vi "UHR-Fleezers Control (host) - 12.3.1.vi"() -> ()   [LabVIEW 2012] (continued)
        n2497 = Add(x=w3700, y=w3699) -> (x+y=w3686:dbl[][])
        n2498 = Add(x=w3674, y=w3673) -> (x+y=w3660:dbl[][])
        n2499 = Add(x=w3768, y=w3767) -> (x+y=w3766:dbl[][])
        n2500 = Add(x=w3772, y=w3771) -> (x+y=w3746:dbl[][])
        n2501 = Add(x=w3754, y=w3753) -> (x+y=w3752:dbl[][])
        n2502 = Add(x=w3761, y=w3760) -> (x+y=w3759:dbl[][])
        n2503 = Divide(x=w3752, y=2) -> (x/y=w3750:dbl[][])
        n2504 = Divide(x=w3766, y=2) -> (x/y=w3711:dbl[][])
        n2505 = To Single Precision Float(number=w3746) -> (single precision float=w3745:sgl[][])
        n2506 = To Single Precision Float(number=w3686) -> (single precision float=w3690:sgl[][])
        n2507 = To Single Precision Float(number=w3660) -> (single precision float=w3664:sgl[][])
        n2508 = Divide(x=w3759, y=2) -> (x/y=w3713:dbl[][])
        n2509 = Transpose 2D Array(2D array=w3750) -> (transposed array=→"Data map":dbl[][])
        n2510 = To Single Precision Float(number=w3711) -> (single precision float=w3717:sgl[][])
        n2511 = To Single Precision Float(number=w3713) -> (single precision float=w3714:sgl[][])
        n2512 = call "IMAQ ArrayToImage"("Image Pixels (Float)"=w3745, "Image"=w3683) -> ("Image Out"=w3748:T2)  [unwired: 8 in, 1 out]
        n2513 = call "IMAQ ArrayToImage"("Image Pixels (Float)"=w3690, "Image"=w3682) -> ("Image Out"=w3692:T2)  [unwired: 8 in, 1 out]
        n2514 = call "IMAQ ArrayToImage"("Image Pixels (Float)"=w3664, "Image"=w3656) -> ("Image Out"=w3666:T2)  [unwired: 8 in, 1 out]
        n2515 = call "IMAQ ArrayToImage"("Image Pixels (Float)"=w3717, "Image"=w3657) -> ("Image Out"=w3719:T2)  [unwired: 8 in, 1 out]
        n2516 = call "IMAQ Symmetry"("Type of Symmetry"=w3747, "Image Src"=w3748) -> ("Image Dst Out"=w3743:T2)  [unwired: 3 in, 1 out]
        n2517 = call "IMAQ ArrayToImage"("Image Pixels (Float)"=w3714, "Image"=w3658) -> ("Image Out"=w3716:T2)  [unwired: 8 in, 1 out]
        n2518 = call "IMAQ Symmetry"("Type of Symmetry"=w3691, "Image Src"=w3692) -> ("Image Dst Out"=w3688:T2)  [unwired: 3 in, 1 out]
        n2519 = call "IMAQ Symmetry"("Type of Symmetry"=w3665, "Image Src"=w3666) -> ("Image Dst Out"=w3662:T2)  [unwired: 3 in, 1 out]
        n2520 = call "IMAQ Symmetry"("Type of Symmetry"=w3718, "Image Src"=w3719) -> ("Image Dst Out"=→"Detection Laser X":T2)  [unwired: 3 in, 1 out]
        n2521 = call "IMAQ Symmetry"("Type of Symmetry"=w3715, "Image Src"=w3716) -> ("Image Dst Out"=→"Detection Laser Y":T2)  [unwired: 3 in, 1 out]
        n2522 = call "IMAQ Set Simple Calibration"("Calibration Axis Info"=T33 {"Origin Pixel"={"X"=0.0, "Y"=0.0}, "Angle Relative to Horizontal (deg)"=0.0, "Axis Reference"=0}, "Grid Descriptor"=T34 {"X Step"=0.3, "Y Step"=0.3, "Unit"=enum."Undefined"}, "Image"=w3743) -> ("Calibrated Image"=→"APD 1":T2)  [unwired: 7 in, 1 out]
        n2523 = call "IMAQ Set Simple Calibration"("Calibration Axis Info"=T33 {"Origin Pixel"={"X"=0.0, "Y"=0.0}, "Angle Relative to Horizontal (deg)"=0.0, "Axis Reference"=0}, "Grid Descriptor"=T34 {"X Step"=0.3, "Y Step"=0.3, "Unit"=enum."Undefined"}, "Image"=w3688) -> ("Calibrated Image"=→"APD 2":T2)  [unwired: 7 in, 1 out]
        n2524 = call "IMAQ Set Simple Calibration"("Calibration Axis Info"=T33 {"Origin Pixel"={"X"=0.0, "Y"=0.0}, "Angle Relative to Horizontal (deg)"=0.0, "Axis Reference"=0}, "Grid Descriptor"=T34 {"X Step"=0.3, "Y Step"=0.3, "Unit"=enum."Undefined"}, "Image"=w3662) -> ("Calibrated Image"=→"APD 3":T2)  [unwired: 7 in, 1 out]
      }
    }
    n2525 = case "For computing FFTs for display" shown="True" "Compute FFT" {
      tunnel: w3158 -> [_ w4286]
      frame False {
      }
      frame True {
        n2526 = Build Array("FFT 1 Choice 1", "FFT 1 Choice 2", "FFT 2 Choice 1", "FFT 2 Choice 2") -> (w4279:u16[])
        n2527 = Array Size(array=w4286) -> (size(s)=w4285:i32)
        n2528 = feedback-in #17(w4279) -> ()
        n2529 = feedback #17(u16[] [100, 100, 100, 100]) -> (w4280:u16[])
        n2530 = feedback-in #18("# Spectra to Ave.") -> ()
        n2531 = feedback #18("# Spectra to Ave.") -> (w4277:dbl)
        n2532 = Not Equal?(x="# Spectra to Ave.", y=w4277) -> (x != y?=w4276:bool)
        n2533 = Not Equal?(x=w4279, y=w4280) -> (x != y?=w4278:bool)
        n2534 = feedback #19(1.0) -> (w4263:dbl)
        n2535 = Compound Arithmetic op=OR("Reset FFT", w4278, w4276) -> (w4261:bool)
        n2536 = Select(t=1.0, s=w4261, f=w4263) -> (s? t:f=w4265:dbl)
        n2537 = Greater?(x=w4265, y="# Spectra to Ave.") -> (0:w4284:bool)
        n2538 = Increment(x=w4265) -> (x+1=w4264:dbl)
        n2539 = feedback-in #19(w4264) -> ()
        n2540 = local read "DMA Update Period (s)"() -> (w4259:dbl)
        n2541 = Multiply(x="# Spectra to Ave.", y=w4259) -> (x*y=→"Ave. Time (s)":dbl)
        n2542 = Build Array(cluster{"f0":dbl, "df":dbl, "magnitude":dbl[]} {"f0"=0.0, "df"=0.0, "magnitude"=[]} ("PSD")) -> (w4268:cluster{"f0":dbl, "df":dbl, "magnitude":dbl[]}[])
        n2543 = Build Array(w4268, w4268, w4268, w4268) -> (w4270:T43)
        n2544 = feedback #20(w4270) -> (w4275:T43)
        n2545 = for {
          N: 4 -> [_]
          tunnel: w4279 -> [w4308] mode=indexing
          tunnel: w4286 -> [w4309]
          tunnel: w4285 -> [w4311]
          tunnel: w4261 -> [w4304]
          tunnel: w4284 -> [w4303]
          tunnel: "# Spectra to Ave." -> [w4302]
          tunnel: [w4301] -> w4274 mode=indexing
          tunnel: w4275 -> [w4306] mode=indexing
          tunnel: [w4305] -> w4262 mode=indexing
          tunnel: w4265 -> [w4300]
          n2546 = Less?(x=w4308, y=w4311) -> (x < y?=w4310:bool)
          n2547 = Index Array(array=w4309, index=w4308) -> (element=w4307:waveform(dbl))
          n2548 = case shown="True" w4310 {
            tunnel: w4307 -> [_ w4328]
            tunnel: w4306 -> [w4313 w4326]
            tunnel: [w4313 w4314] -> w4305
            tunnel: w4304 -> [_ w4325]
            tunnel: w4303 -> [_ w4318]
            tunnel: w4302 -> [_ w4317]
            tunnel: [cluster{"f0":dbl, "df":dbl, "magnitude":dbl[]} {"f0"=0.0, "df"=0.0, "magnitude"=[]} ("PSD") w4319] -> w4301
            tunnel: w4300 -> [_ w4316]
            frame False {
            }
            frame True {
              n2549 = call <vilib>:"Std Deviation and Variance.vi"("X"=w4328) -> ("mean"=w4329:dbl)  [unwired: 1 in, 2 out]
              n2550 = Subtract(x=w4328, y=w4329) -> (x-y=w4327:waveform(dbl))
              n2551 = xnode "Spectral Measurements"("Signals"=w4327) -> ("PSD"=w4321:cluster{"f0":dbl, "df":dbl, "magnitude":dbl[]})  [unwired: 1 in, 1 out]
              n2552 = case shown="False" w4325 {
                tunnel: w4326 -> [w4338 _]
                tunnel: [w4334 w4343] -> w4314
                tunnel: w4321 -> [w4337 w4344]
                tunnel: w4318 -> [w4336 _]
                frame False {
                  n2553 = Build Array (concatenate)(w4338, w4337) -> (w4335:cluster{"f0":dbl, "df":dbl, "magnitude":dbl[]}[])
                  n2554 = case shown="True" w4336 {
                    tunnel: w4335 -> [w4339 w4342]
                    tunnel: [w4339 w4340] -> w4334
                    frame False {
                    }
                    frame True {
                      n2555 = Delete From Array(array=w4342, index=0) -> (array with subset deleted=w4340:cluster{"f0":dbl, "df":dbl, "magnitude":dbl[]}[])  [unwired: 1 in, 1 out]
                    }
                  }
                }
                frame True {
                  n2556 = Build Array(w4344) -> (w4343:cluster{"f0":dbl, "df":dbl, "magnitude":dbl[]}[])
                }
              }
              n2557 = for {
                tunnel: w4314 -> [w4333] mode=indexing
                tunnel: [w4332] -> w4324 mode=indexing
                workers-P: _ -> [_]
                n2558 = Unbundle By Name(w4333) -> ("magnitude"=w4332:dbl[])
              }
              n2559 = Transpose 2D Array(2D array=w4324) -> (transposed array=w4323:dbl[][])
              n2560 = for {
                tunnel: w4323 -> [w4331] mode=indexing
                tunnel: [w4330] -> w4322 mode=indexing
                workers-P: _ -> [_]
                n2561 = Add Array Elements(numeric array=w4331) -> (sum=w4330:dbl)
              }
              n2562 = Select(t=w4317, s=w4318, f=w4316) -> (s? t:f=w4315:dbl)
              n2563 = Divide(x=w4322, y=w4315) -> (x/y=w4320:dbl[])
              n2564 = Bundle By Name(cluster=w4321, "magnitude"=w4320) -> (w4319:cluster{"f0":dbl, "df":dbl, "magnitude":dbl[]})
            }
          }
        }
        n2565 = case shown="True" w4261 {
          tunnel: w4262 -> [w4293 w4299]
          tunnel: [w4293 w4294] -> w4260
          frame False {
          }
          frame True {
            n2566 = Array Subset(array=w4299, index (row)=0 ("index"), length (row)=4 ("length"), index (col)=0 ("index"), length (col)=1 ("length")) -> (w4294:T43)
          }
        }
        n2567 = feedback-in #20(w4260) -> ()
        n2568 = Split 1D Array(array=w4274, index=2) -> (first subarray=→"FFT 1":cluster{"f0":dbl, "df":dbl, "magnitude":dbl[]}[], second subarray=→"FFT 2":cluster{"f0":dbl, "df":dbl, "magnitude":dbl[]}[])
      }
    }
    n2569 = Index Array(array=w3156, index=4) -> (element=w3212:waveform(dbl))
    n2570 = Index Array(array=w3156, index=7) -> (element=w3209:waveform(dbl))
    n2571 = Divide(x="T1 offset_x (mV)", y=1000.0) -> (x/y=w3213:dbl)
    n2572 = feedback-in #21("Calibration") -> ()
    n2573 = feedback #21(u16 1 ("Calibration")) -> (w3231:u16)
    n2574 = Divide(x="T2 offset_x (mV)", y=1000.0) -> (x/y=w3211:dbl)
    n2575 = case shown="2" "Calibration" {
      tunnel: "T1 alpha_x (nm/V)" -> [_ w3607 w3628]
      tunnel: "T1 kappa_x (pN/nm)" -> [_ _ w3618]
      tunnel: "T2 alpha_x (nm/V)" -> [_ w3606 w3626]
      tunnel: "T2 kappa_x (pN/nm)" -> [_ _ w3619]
      tunnel: w3212 -> [w3589 w3604 w3624]
      tunnel: w3209 -> [w3588 w3602 w3622]
      tunnel: [w3589 w3601 w3621] -> w3240
      tunnel: [w3588 w3600 w3620] -> w3239
      tunnel: ["T1 X (V)" ("Label.Text") "T1 X (nm)" ("Label.Text") "T1 X (pN)" ("Label.Text")] -> w3228
      tunnel: ["T2 X (V)" ("Label.Text") "T2 X (nm)" ("Label.Text") "T2 X (pN)" ("Label.Text")] -> w3227
      tunnel: ["Position (V)" ("Label.Text") "Position (nm)" ("Label.Text") "Force (pN)" ("Label.Text")] -> w3229
      tunnel: w3211 -> [_ w3592 w3611]
      tunnel: w3213 -> [_ w3595 w3613]
      tunnel: ["Mean (V)" ("Label.Text") "Mean (nm)" ("Label.Text") "Mean (pN)" ("Label.Text")] -> w3224
      tunnel: ["Difference (V)" ("Label.Text") "Difference (nm)" ("Label.Text") "Difference (pN)" ("Label.Text")] -> w3164
      frame 0, Default {
      }
      frame 1 {
        n2576 = Unbundle By Name(w3604) -> ("Y"=w3608:dbl[])
        n2577 = Unbundle By Name(w3602) -> ("Y"=w3593:dbl[])
        n2578 = Subtract(x=w3608, y=w3595) -> (x-y=w3596:dbl[])
        n2579 = Subtract(x=w3593, y=w3592) -> (x-y=w3594:dbl[])
        n2580 = Multiply(x=w3594, y=w3606) -> (x*y=w3603:dbl[])
        n2581 = Multiply(x=w3607, y=w3596) -> (x*y=w3605:dbl[])
        n2582 = Bundle By Name(cluster=w3602, "Y"=w3603) -> (w3600:waveform(dbl))
        n2583 = Bundle By Name(cluster=w3604, "Y"=w3605) -> (w3601:waveform(dbl))
      }
      frame 2 {
        n2584 = Unbundle By Name(w3624) -> ("Y"=w3629:dbl[])
        n2585 = Unbundle By Name(w3622) -> ("Y"=w3627:dbl[])
        n2586 = Subtract(x=w3627, y=w3611) -> (x-y=w3612:dbl[])
        n2587 = Subtract(x=w3629, y=w3613) -> (x-y=w3614:dbl[])
        n2588 = Compound Arithmetic op=MULTIPLY(w3612, w3626, w3619) -> (w3623:dbl[])
        n2589 = Compound Arithmetic op=MULTIPLY(w3618, w3628, w3614) -> (w3625:dbl[])
        n2590 = Bundle By Name(cluster=w3622, "Y"=w3623) -> (w3620:waveform(dbl))
        n2591 = Bundle By Name(cluster=w3624, "Y"=w3625) -> (w3621:waveform(dbl))
      }
    }
    n2592 = case shown="True" "Read Lateness and Rel Phase" {
      tunnel: w3030 -> [w3538 w3577]
      tunnel: w3029 -> [w3539 w3576]
      tunnel: [w3538 w3543] -> w3206
      tunnel: [w3539 w3542] -> w3205
      frame False {
      }
      frame True {
        n2593 = xnode "Read/Write Control"("FPGA VI Reference In"=w3577, "error in"=w3576) -> ("FPGA VI Reference Out"=w3545:T19, "error out"=w3544:errorcluster, "GI Relative phase"=→"GI relative phase":i16, "Relative phase"=→"Relative phase (AI1)":i16, "AI Late Counter"=→"Late Counter (AI1)":u8, "GI Late Counter"=→"GI Late Counter":u8, "MCL Late Counter"=→"MCL Late Counter":u8, "MCL Relative Phase"=→"Relative Phase (MCL)":i16, "APD Acq Relative Phase"=→"APD Acq Relative Phase":i16, "APD 1 Gate Relative Phase"=→"APD 1 Gate Relative Phase":i16, "APD 2 Gate Relative Phase"=→"APD 2 Gate Relative Phase":i16, "APD Acq Late Counter"=→"APD Acq Late Counter":u8, "APD 1 Gate Late Counter"=→"APD 1 Gate Late Counter":u8, "APD 2 Gate Late Counter"=→"APD 2 Gate Late Counter":u8, "Green FB Relative Phase"=→"Relative phase (Green FB)":i16, "GI Relative phase 2"=→"GI relative phase 2":i16, "GI Late Counter 2"=→"GI Late Counter 2":u8, "Trap Pos FIFO Timeout"=→"Trap Pos FIFO Timeout":u16, "Trap AI FIFO Timeout"=→"Trap AI FIFO Timeout":u16, "RI Late Counter"=→"RI Late Counter":u8, "RI Late Counter 2"=→"RI Late Counter 2":u8, "RI Relative phase"=→"RI relative phase":i16, "RI Relative phase 2"=→"RI relative phase 2":i16, "Red FB Relative Phase"=→"Relative phase (RI FB)":i16, "Red Late Counter"=→"Red AI Late Counter":u8, "Green Late Counter"=→"Green AI Late Counter":u8, "BI Late Counter (AO)"=→"Late Counter (BI AO)":u8, "Blue Late Counter (D)"=→"Late Counter (BI DO)":u8, "Blue Int Late Counter"=→"Late Counter (BI AI)":u8, "Blue Int Relative Phase"=→"Relative phase (BI AI)":i16, "BI Relative phase (AO)"=→"Relative phase (BI AO)":i16, "BI Relative phase (D)"=→"Relative phase (BI DO)":i16)
        n2594 = xnode "Read/Write Control"("FPGA VI Reference In"=w3545, "error in"=w3544) -> ("FPGA VI Reference Out"=w3543:T19, "error out"=w3542:errorcluster, "APD 3 Gate Late Counter"=→"APD 3 Gate Late Counter":u8, "APD 3 Gate Relative Phase"=→"APD 3 Gate Relative Phase":i16)
      }
    }
    n2595 = Not Equal?(x=w3231, y="Calibration") -> (x != y?=w3190:bool)
    n2596 = case shown="True" w3190 {
      tunnel: w3229 -> [_ w3582]
      tunnel: w3228 -> [_ w3581]
      tunnel: w3227 -> [_ w3580]
      tunnel: w3224 -> [_ w3579]
      tunnel: w3164 -> [_ w3578]
      frame False {
      }
      frame True {
        n2597 = property on="Force" class="WFChart (strict)"("YScale.NameLbl.Text"=w3582) -> ()  [unwired: 2 in, 2 out]
        n2598 = property on="T2 X" class="DigNum (strict)"("Caption.Text"=w3580) -> ()  [unwired: 2 in, 2 out]
        n2599 = property on="T1 X" class="DigNum (strict)"("Caption.Text"=w3581) -> ()  [unwired: 2 in, 2 out]
        n2600 = property on="Mean" class="DigNum (strict)"("Caption.Text"=w3579) -> ()  [unwired: 2 in, 2 out]
        n2601 = property on="Difference" class="DigNum (strict)"("Caption.Text"=w3578) -> ()  [unwired: 2 in, 2 out]
      }
    }
    n2602 = Unbundle By Name(w3212) -> ("Y"=w3215:dbl[])
    n2603 = Unbundle By Name(w3209) -> ("Y"=w3218:dbl[])
    n2604 = Subtract(x=w3215, y=w3213) -> (x-y=w3216:dbl[])
    n2605 = Subtract(x=w3218, y=w3211) -> (x-y=w3217:dbl[])
    n2606 = Multiply(x=w3217, y="T2 alpha_x (nm/V)") -> (x*y=w3012:dbl[])
    n2607 = Multiply(x="T1 alpha_x (nm/V)", y=w3216) -> (x*y=w3013:dbl[])
    n2608 = Not(x="Trap Trig. Fl.") -> (.not. x?=w3049:bool)
    n2609 = Multiply(x=w3239, y=-1.0) -> (x*y=w3220:waveform(dbl))
    n2610 = Subtract(x=w3013, y=w3012) -> (x-y=w3208:dbl[])
    n2611 = Unbundle By Name(w3239) -> ("Y"=w3180:dbl[])
    n2612 = Unbundle By Name(w3240) -> ("Y"=w3014:dbl[])
    n2613 = Negate(x=w3208) -> (-x=w3010:dbl[])
    n2614 = Build Array(w3240, w3220) -> (→"Force":waveform(dbl)[])
    n2615 = Subtract(x=w3010, y="Offset (nm)") -> (x-y=w3178:dbl[])
    n2616 = call-poly <vilib>:"Mean.vi"("X"=w3180) -> ("mean"=w3016:dbl)  [unwired: 1 out]
    "T2 X" <- w3016
    n2617 = Negate(x=w3180) -> (-x=w3181:dbl[])
    n2618 = call-poly <vilib>:"Mean.vi"("X"=w3014) -> ("mean"=w3017:dbl)  [unwired: 1 out]
    "T1 X" <- w3017
    n2619 = Negate(x=w3016) -> (-x=w3015:dbl)
    n2620 = Bundle By Name(cluster=w3212, "Y"=w3178) -> (w3155:waveform(dbl))
    "Bead Separation" <- w3155
    n2621 = Add(x=w3014, y=w3181) -> (x+y=w3182:dbl[])
    n2622 = Add(x=w3017, y=w3015) -> (x+y=w3226:dbl)
    n2623 = Subtract(x=w3017, y=w3015) -> (x-y=→"Difference":dbl)
    n2624 = Divide(x=w3182, y=2.0) -> (x/y=→"Vec Mean of T1 T2":dbl[])
    n2625 = Divide(x=w3226, y=2.0) -> (x/y=w3184:dbl)
    "Mean" <- w3184
    n2626 = feedback-in #22("Trap Trig. Fl.") -> ()
    n2627 = feedback #22("Trap Trig. Fl.") -> (w3047:bool)
    n2628 = And(x=w3049, y=w3047) -> (x .and. y?=w3048:bool)
    n2629 = case "If have just turned off triggering" shown="True" w3048 {
      tunnel: w3030 -> [_ w3373]
      tunnel: w3029 -> [_ w3372]
      frame False {
      }
      frame True {
        w3371 = FALSE ("FPGA Trap Trig")
        n2630 = xnode "Read/Write Control"("FPGA VI Reference In"=w3373, "error in"=w3372, "FPGA Trap Trig"=w3371) -> ("FPGA VI Reference Out"=w3370:T19, "error out"=w3369:errorcluster)
        n2631 = xnode "Read/Write Control"("FPGA VI Reference In"=w3370, "error in"=w3369, "TTrig?"=w3371) -> ()  [unwired: 2 out]
        n2632 = local write "Initializing"(FALSE ("Initializing")) -> ()
        n2633 = local write "Triggered"(FALSE ("Triggered")) -> ()
        n2634 = local write "Waiting"(FALSE ("Waiting")) -> ()
      }
    }
    n2635 = Not(x=w3047) -> (.not. x?=w3060:bool)
    n2636 = And(x="Trap Trig. Fl.", y=w3060) -> (x .and. y?=w3057:bool)
    n2637 = local read "Tether"() -> (w3185:bool)
    n2638 = Or(x=w3057, y="Reinitialize") -> (x .or. y?=w3043:bool)
    n2639 = feedback #23(w3053) -> (w3058:string)
    n2640 = Select(t=w3053, s=w3057, f=w3058) -> (s? t:f=w3052:string)
    n2641 = Select(t=w3053, s="Reinitialize", f=w3052) -> (s? t:f=w3051:string)
    n2642 = feedback #24(0) -> (w3055:i32)
    n2643 = feedback #25(w3178) -> (w3177:dbl[])
    n2644 = Build Array (concatenate)(w3178, w3177) -> (w3011:dbl[])
    n2645 = case "For determining if there is a tether still" shown="True" w3185 {
      tunnel: w3184 -> [_ w3497]
      frame False {
      }
      frame True {
        n2646 = Greater?(x="Lost Tether Alarm Threshold (pN)", y=w3497) -> (0:w3495:bool)
        n2647 = case shown="True" w3495 {
          frame False {
          }
          frame True {
            w3498 = FALSE ("Value (Signaling)")
            n2648 = flat-sequence {
              frame #0 {
                # "stop only if saving"
                n2649 = local read "Saving..."() -> (w3510:bool)
                n2650 = And(x=w3510, y="TA Cancel Save?") -> (x .and. y?=w3509:bool)
                n2651 = local write "Stop Saving"(w3509) -> ()
              }
              frame #1 {
                n2652 = case shown="True" "TA Green Off?" {
                  frame False {
                  }
                  frame True {
                    w3513 = FALSE ("Fl. Triggered...")
                    n2653 = local write "Fl. Triggered..."(w3513) -> ()
                    n2654 = property on="Green Laser ON" class="Bool (strict)"("Val(Sgnl)"=w3513) -> ()  [unwired: 2 in, 2 out]
                  }
                }
              }
            }
            n2655 = local read "Time tether formed"() -> (w3504:timestamp)
            n2656 = Get Date/Time In Seconds() -> (seconds since 1Jan1904=w3505:timestamp)
            n2657 = Subtract(x=w3505, y=w3504) -> (x-y=w3503:dbl)
            n2658 = Number To Decimal String(number=w3503) -> (decimal integer string=w3500:string)  [unwired: 1 out]
            n2659 = local read "Messages"() -> (w3507:string)
            n2660 = call <vilib>:"Beep.vi"() -> ()  [unwired: 3 in, 9 out]
            n2661 = Concatenate Strings("Lost tether (" ("Message to add"), w3500, " s)." ("string")) -> (w3502:string)
            n2662 = local write "Tether"(FALSE ("Tether")) -> ()
            n2663 = call "Update messages.vi"("Message to add"=w3502, "Old message string"=w3507) -> ("New message string"=w3506:string)
            n2664 = local write "Messages"(w3506) -> ()
            n2665 = property on="Fl. Triggered..." class="Bool (strict)"("Val(Sgnl)"=w3498) -> ()  [unwired: 2 in, 2 out]
            n2666 = local write "Dip for Protein"(w3498) -> ()
            n2667 = property on="Trap Pos. FB ON" class="Bool (strict)"("Val(Sgnl)"=w3498) -> ()  [unwired: 2 in, 2 out]
            n2668 = property on="Trap Trig. Fl." class="Bool (strict)"("Val(Sgnl)"=w3498) -> ()  [unwired: 2 in, 2 out]
          }
        }
      }
    }
    n2669 = case "For triggering actions based on the trap position (e.g., turning the excitation laser on if trap under feedback moves so far)" shown="True" "Trap Trig. Fl." {
      tunnel: w3038 -> [_ w3386]
      tunnel: w3051 -> [_ w3385]
      tunnel: ["" ("t") w3384] -> w3059
      tunnel: w3043 -> [_ w3383]
      tunnel: [0 ("t") w3382] -> w3056
      tunnel: w3055 -> [_ w3381]
      tunnel: w3030 -> [_ w3380]
      tunnel: w3029 -> [_ w3379]
      frame False {
      }
      frame True {
        n2670 = case shown="\"Wait for trigger\"" w3385 {
          tunnel: w3386 -> [w3403 _ _ w3451]
          tunnel: [w3400 w3432 "" ("t") w3454] -> w3384
          tunnel: w3383 -> [_ _ _ w3442]
          tunnel: [w3399 w3429 0 ("t") w3443] -> w3382
          tunnel: w3381 -> [_ w3431 _ w3449]
          tunnel: w3380 -> [w3388 w3426 _ w3445]
          tunnel: w3379 -> [w3387 w3425 _ w3444]
          frame "Wait for trigger" {
            n2671 = local read "Trap Trig. (FPGA)"() -> (w3391:bool)
            n2672 = Subtract(x=w3403, y="Mean T1 Position\nto compare (nm)") -> (x-y=w3396:dbl[])
            n2673 = call <vilib>:"Std Deviation and Variance.vi"("X"=w3396) -> ("mean"=→"mean":dbl, "standard deviation"=→"standard\ndeviation":dbl)  [unwired: 1 in, 1 out]
            n2674 = Array Max & Min(array=w3396) -> (max value=→"max value":dbl, min value=→"min value":dbl)  [unwired: 2 out]
            n2675 = Greater?(x=w3396, y="Threshold (nm)") -> (0:w3406:bool[])
            n2676 = case shown="True" w3391 {
              tunnel: w3388 -> [_ w3412]
              tunnel: w3387 -> [_ w3411]
              tunnel: [FALSE ("TTrig?") w3410] -> w3394
              frame False {
              }
              frame True {
                n2677 = xnode "Read/Write Control"("FPGA VI Reference In"=w3412, "error in"=w3411) -> ("TTrig?"=w3410:bool)  [unwired: 2 out]
              }
            }
            n2678 = Or Array Elements(Boolean array=w3406) -> (logical OR=w3393:bool)
            n2679 = Select(t=w3394, s=w3391, f=w3393) -> (s? t:f=w3392:bool)
            n2680 = Not(x=w3391) -> (.not. x?=w3390:bool)
            n2681 = And(x=w3392, y=w3390) -> (x .and. y?=w3389:bool)
            n2682 = Select(t="Triggered", s=w3392, f="Wait for trigger") -> (s? t:f=w3400:string)
            n2683 = case shown="True" w3392 {
              tunnel: [0 0] -> w3399
              tunnel: w3388 -> [_ w3417]
              tunnel: w3387 -> [_ w3416]
              frame False {
                "Waiting" <- TRUE ("Waiting")
              }
              frame True {
                n2684 = xnode "Read/Write Control"("FPGA VI Reference In"=w3417, "error in"=w3416, "TTrig?"=FALSE) -> ()  [unwired: 2 out]
                n2685 = local read "Messages"() -> (w3420:string)
                n2686 = call <vilib>:"Beep.vi"() -> ()  [unwired: 12 in]
                n2687 = call "Update messages.vi"("Message to add"="Unwinding trigger.", "Old message string"=w3420) -> ("New message string"=w3421:string)
                n2688 = local write "Messages"(w3421) -> ()
                n2689 = local write "Waiting"(FALSE ("Waiting")) -> ()
                "Triggered" <- TRUE ("Triggered")
              }
            }
            n2690 = case "Only need to turn on laser if host triggered" shown="True" w3389 {
              frame False {
              }
              frame True {
                n2691 = property on="Green Laser ON" class="Bool (strict)"("Val(Sgnl)"=TRUE ("Value (Signaling)")) -> ()  [unwired: 2 in, 2 out]
              }
            }
          }
          frame "Triggered" {
            n2692 = local read "Trap Trig. (FPGA)"() -> (w3428:bool)
            n2693 = Increment(x=w3431) -> (x+1=w3429:i32)
            n2694 = Greater Or Equal?(x=w3429, y="Fl. ON time (n)") -> (x >= y?=w3427:bool)
            n2695 = Select(t="Wait for trigger", s=w3427, f="Triggered" ("t")) -> (s? t:f=w3432:string)
            n2696 = And(x=w3427, y=w3428) -> (x .and. y?=w3424:bool)
            n2697 = case shown="True" w3424 {
              tunnel: w3426 -> [_ w3436]
              tunnel: w3425 -> [_ w3435]
              frame False {
              }
              frame True {
                n2698 = xnode "Read/Write Control"("FPGA VI Reference In"=w3436, "error in"=w3435, "FPGA Trap Trig"=TRUE) -> ()  [unwired: 2 out]
              }
            }
            n2699 = case shown="True" w3427 {
              frame False {
              }
              frame True {
                w3438 = FALSE ("Value (Signaling)")
                n2700 = local write "Triggered"(w3438) -> ()
                n2701 = local write "Waiting"(TRUE ("Waiting")) -> ()
                n2702 = property on="Green Laser ON" class="Bool (strict)"("Val(Sgnl)"=w3438) -> ()  [unwired: 2 in, 2 out]
              }
            }
          }
          frame "Do nothing" {
          }
          frame "Initialize", Default {
            n2703 = Increment(x=w3449) -> (x+1=w3453:i32)
            n2704 = Select(t=1, s=w3442, f=w3453) -> (s? t:f=w3443:i32)
            n2705 = feedback #26(w3451) -> (w3457:dbl[])
            n2706 = Build Array (concatenate)(w3451, w3457) -> (w3450:dbl[])
            n2707 = Greater Or Equal?(x=w3443, y="Wait to get offset (n)") -> (x >= y?=w3446:bool)
            n2708 = Select(t=w3451, s=w3442, f=w3450) -> (s? t:f=w3452:dbl[])
            n2709 = feedback-in #26(w3452) -> ()
            n2710 = call-poly <vilib>:"Mean.vi"("X"=w3452) -> ("mean"=w3447:dbl)  [unwired: 1 out]
            n2711 = local write "Mean T1 Position\nto compare (nm)"(w3447) -> ()
            n2712 = case shown="True" w3442 {
              tunnel: w3445 -> [_ w3463]
              tunnel: w3444 -> [_ w3462]
              frame False {
              }
              frame True {
                w3459 = FALSE ("FPGA Trap Trig")
                n2713 = xnode "Read/Write Control"("FPGA VI Reference In"=w3463, "error in"=w3462, "FPGA Trap Trig"=w3459) -> ("FPGA VI Reference Out"=w3461:T19, "error out"=w3460:errorcluster)
                n2714 = xnode "Read/Write Control"("FPGA VI Reference In"=w3461, "error in"=w3460, "TTrig?"=w3459) -> ()  [unwired: 2 out]
              }
            }
            n2715 = Select(t="Wait for trigger", s=w3446, f="Initialize") -> (s? t:f=w3454:string)
            n2716 = case shown="True" w3446 {
              tunnel: w3447 -> [_ w3466]
              tunnel: w3445 -> [_ w3475]
              tunnel: w3444 -> [_ w3474]
              frame False {
                n2717 = local write "Waiting"(FALSE ("Waiting")) -> ()
                "Initializing" <- TRUE ("Initializing")
              }
              frame True {
                n2718 = local read "Threshold (nm)"() -> (w3478:dbl)
                n2719 = local read "AOM X Cal (nm/MHz)"() -> (w3477:dbl)
                n2720 = Add(x=w3466, y=w3478) -> (x+y=w3479:dbl)
                n2721 = Divide(x=w3479, y=w3477) -> (x/y=w3476:dbl)
                n2722 = call "IR AOM freq to word.vi"("Frequency In (MHz)"=w3476) -> ("Frequency Word Out (double)"=w3473:dbl)
                n2723 = local write "Initializing"(FALSE ("Initializing")) -> ()
                n2724 = local write "Waiting"(TRUE ("Waiting")) -> ()
                n2725 = To Quad Integer(1:w3473) -> (0:w3472:i64)
                n2726 = xnode "Read/Write Control"("FPGA VI Reference In"=w3475, "error in"=w3474, "FPGA TTrig Thresh"=w3472) -> ("FPGA VI Reference Out"=w3469:T19, "error out"=w3468:errorcluster)
                n2727 = xnode "Read/Write Control"("FPGA VI Reference In"=w3469, "error in"=w3468, "FPGA Trap Trig"=TRUE) -> ()  [unwired: 2 out]
              }
            }
          }
        }
      }
    }
    n2728 = feedback-in #23(w3059) -> ()
    n2729 = feedback-in #24(w3056) -> ()
    n2730 = Split 1D Array(array=w3011, index=w3073) -> (first subarray=w3174:dbl[])  [unwired: 1 out]
    n2731 = feedback-in #25(w3174) -> ()
    n2732 = call-poly <vilib>:"Mean.vi"("X"=w3174) -> ("mean"=w3173:dbl)  [unwired: 1 out]
    "Bead Mean (nm)" <- w3173
    n2733 = Subtract(x=w3174, y=w3173) -> (x-y=w3172:dbl[])
    n2734 = Square(x=w3172) -> (x^2=w3171:dbl[])
    n2735 = call-poly <vilib>:"Mean.vi"("X"=w3171) -> ("mean"=w3170:dbl)  [unwired: 1 out]
    n2736 = Square Root(x=w3170) -> (sqrt(x)=w3169:dbl)
    n2737 = Multiply(x=10.0, y=w3169) -> (x*y=→"RMS (Ang)":dbl)
    n2738 = xnode ("Read/Write Control")("FPGA VI Reference In"=w3206, "error in"=w3205) -> ("FPGA VI Reference Out"=w3041:T19, "error out"=w3040:errorcluster, "AI2 Y Sum Set 1"=w3304:i16, "AI2 Y Sum Set 2"=w3303:i16, "AI1 X Set 1"=w3105:fxp<+/-,16,1>, "AI1 X Set 2"=w3104:fxp<+/-,16,1>, "Trap Pos FB Int Signal"=→"Trap Pos FB Int Signal":fxp<+/-,24,9>, "Trap Pos FB Int-Norm Signal"=→"Trap Pos FB Int-Norm Signal":fxp<+/-,16,1>, "Trap Pos FB Action"=w3098:i64, "Scanning"=→"AOD Scanning":bool, "Scan I"=→"AOD Scan I":u64, "Scanning MCL"=w3306:bool, "Scan I (MCL)"=→"MCL Scan I":u64, "Green FB Sum"=w3243:i16, "Trap Pos FB Action"=w3028:i64, "TTrig Fin Thresh"=w3024:i64, "Red FB Intensity"=w3005:i16, "Blue Intensity"=w3000:i16)
    "MCL Scanning" <- w3306
    "Trap Pos FB Action" <- w3098
    n2739 = Divide(x=w3005, y=3276.7) -> (x/y=w3004:dbl)
    "Red laser intensity (V)" <- w3004
    n2740 = Divide(x=w3000, y=3276.7) -> (x/y=w2999:dbl)
    "Blue laser intensity (V)" <- w2999
    n2741 = Divide(x=w3243, y=3276.7) -> (x/y=w3003:dbl)
    "Green laser intensity (V)" <- w3003
    n2742 = local read "FB Trig Integrate"() -> (w3022:u32)
    n2743 = Divide(x=w3028, y=w3022) -> (x/y=w3021:dbl)
    "TTrig Sig (Int)" <- w3021
    n2744 = Bundle(w3003, w3004, w2999) -> (→"Fluorescence laser intensities plot":cluster{dbl, dbl, dbl})  [unwired: 1 in]
    n2745 = Divide(x=w3024, y=w3022) -> (x/y=w3019:dbl)
    "TTrig Fin Thresh (Int)" <- w3019
    n2746 = local read "AOM X Cal (nm/MHz)"() -> (w3027:dbl)
    n2747 = local read "AI2 (V)"() -> (w3305:cluster{"Set 1":dbl, "Set 2":dbl})
    n2748 = Bundle By Name(cluster=w3305, "Set 1"=w3304, "Set 2"=w3303) -> (w3301:cluster{"Set 1":dbl, "Set 2":dbl})
    n2749 = Divide(x=w3098, y=327.67) -> (x/y=→"Action (%)":dbl)
    n2750 = local read "Trap X (AI1)"() -> (w3118:T10)
    n2751 = call "IR AOM word double to freq.vi"("Frequency Word In (double)"=w3019) -> ("Frequency Out (MHz)"=w3018:dbl)
    n2752 = call "IR AOM word double to freq.vi"("Frequency Word In (double)"=w3021) -> ("Frequency Out (MHz)"=w3020:dbl)
    n2753 = Divide(x=w3301, y=3276.7) -> (x/y=w3300:cluster{"Set 1":dbl, "Set 2":dbl})
    n2754 = Multiply(x=w3020, y=w3027) -> (x*y=w3026:dbl)
    "TTrig Sig (nm)" <- w3026
    n2755 = Multiply(x=w3018, y=w3027) -> (x*y=w3025:dbl)
    "TTrig Fin Thresh (nm)" <- w3025
    n2756 = local write "AI2 (V)"(w3300) -> ()
    n2757 = Bundle(cluster=w3118, "Trap 1"=w3105, "Trap 2"=w3104) -> (→"Trap X (AI1)":T10)
    n2758 = Bundle(w3026, w3025) -> (→"TTrig":cluster{dbl, dbl})  [unwired: 1 in]
    n2759 = flat-sequence "To save data" {
      tunnel: [w4392] -> w3324
      tunnel: [w4393] -> w3323
      tunnel: w3274 -> [w4386]
      tunnel: w3046 -> [w4390]
      tunnel: ["Save Calibration"] -> w3297
      tunnel: w3294 -> [w4389]
      tunnel: [w4382] -> w3293
      tunnel: [w4379] -> w3292
      tunnel: [w4376] -> w3291
      tunnel: w3273 -> [w4378]
      tunnel: w3188 -> [w4372]
      tunnel: [w4372] -> w3187
      tunnel: ["Start Saving"] -> w3157
      tunnel: [w4366] -> w3086
      tunnel: [w4365] -> w3085
      tunnel: w3324 -> [w4629]
      tunnel: w3323 -> [w4628]
      tunnel: w3087 -> [w4627]
      tunnel: w3297 -> [w4626]
      tunnel: w3293 -> [w4624]
      tunnel: w3292 -> [w4623]
      tunnel: w3291 -> [w4622]
      tunnel: w3166 -> [w4621]
      tunnel: w3198 -> [w4620]
      tunnel: w3187 -> [w4619]
      tunnel: w3157 -> [w4618]
      tunnel: w3155 -> [w4617]
      tunnel: w2986 -> [w4616]
      tunnel: w3086 -> [w4615]
      tunnel: w3085 -> [w4614]
      tunnel: w3084 -> [w4613]
      tunnel: w3007 -> [w4612]
      frame #0 {
        n2760 = Or(x="Save N Sets", y="Start Saving") -> (x .or. y?=w4373:bool)
        n2761 = To Double Precision Float(number=w4389) -> (double precision float=w4383:dbl)
        n2762 = Build Array(w4373, "Save Calibration", w4386, w4378) -> (w4388:bool[])
        n2763 = Compound Arithmetic op=OR("Save Calibration", w4386, w4373, w4378) -> (w4391:bool)
        n2764 = Boolean Array To Number(Boolean array=w4388) -> (number=w4385:u32)
        n2765 = feedback #27(FALSE ("Save APD Data\nwith Trap Data")) -> (w4367:bool)
        n2766 = feedback #28(refnum<k0> refnum) -> (w4394:refnum<file>)
        n2767 = feedback #29(refnum<k0> refnum) -> (w4369:refnum<file>)
        n2768 = feedback #30(FALSE ("Save APD Data\nwith Trap Data")) -> (w4377:bool)
        n2769 = feedback #31(refnum<k0> refnum) -> (w4380:refnum<file>)
        n2770 = feedback #32(0) -> (w4396:i32)
        n2771 = feedback #33() -> (w4384:u32)  [unwired: 1 out]
        n2772 = case shown="True" w4391 {
          tunnel: [w4403 1] -> w4392
          tunnel: w4396 -> [w4405 _]
          tunnel: [w4404 w4423] -> w4393
          tunnel: w4394 -> [w4404 _]
          tunnel: w4390 -> [_ w4443]
          tunnel: w4383 -> [_ w4441]
          tunnel: w4385 -> [_ w4444]
          tunnel: [w4402 w4422] -> w4382
          tunnel: w4384 -> [w4402 _]
          tunnel: [w4401 w4420] -> w4379
          tunnel: w4380 -> [w4401 _]
          tunnel: [w4400 w4419] -> w4376
          tunnel: w4377 -> [w4400 _]
          tunnel: "Start Saving" -> [_ w4417]
          tunnel: w4372 -> [_ w4416]
          tunnel: [w4399 w4407] -> w4365
          tunnel: w4369 -> [w4399 _]
          tunnel: [w4398 w4406] -> w4366
          tunnel: w4367 -> [w4398 _]
          frame False {
            n2773 = Increment(x=w4405) -> (x+1=w4403:i32)
          }
          frame True {
            w4413 = FALSE ("Start Saving")
            w4418 = 9.0  # File Version
            w4426 = FALSE ("prepend array or string size? (T)")
            w4424 = T25."big-endian, network order" ("byte order (0:big-endian, network order)")
            n2774 = local read "BD 1 Frequency 1 (MHz)"() -> (w4440:dbl)
            n2775 = local read "BD 2 Frequency 1 (MHz)"() -> (w4439:dbl)
            n2776 = local read "BD 1 Frequency 2 (MHz)"() -> (w4438:dbl)
            n2777 = local read "BD 2 Frequency 2 (MHz)"() -> (w4437:dbl)
            n2778 = local read "BD 1 Frequency 3 (MHz)"() -> (w4436:dbl)
            n2779 = local read "BD 2 Frequency 3 (MHz)"() -> (w4435:dbl)
            n2780 = Array Size(array=w4416) -> (size(s)=w4415:i32)
            n2781 = To Double Precision Float(number=w4415) -> (double precision float=w4414:dbl)
            n2782 = local write "Save Calibration"(w4413) -> ()
            n2783 = local write "Start Saving"(w4413) -> ()
            n2784 = Build Array("Save APD Data\nwith Trap Data", "Save Trap Pos. Data") -> (w4410:bool[])
            n2785 = Boolean Array To Number(Boolean array=w4410) -> (number=w4409:u32)
            n2786 = Build Array(w4440, w4439, w4438, w4437, w4436, w4435) -> (w4434:dbl[])
            n2787 = case shown="1, Default" w4444 {
              tunnel: w4443 -> [w4516 w4536 w4552 w4590]
              tunnel: w4414 -> [w4521 w4543 w4572 w4609]
              tunnel: w4441 -> [w4520 w4542 w4571 w4608]
              tunnel: [w4517 w4538 w4563 w4600] -> w4432
              tunnel: [w4508 "Cal sets to save" w4553 w4591] -> w4422
              tunnel: w4434 -> [w4518 w4539 w4565 w4602]
              tunnel: "Save APD Data\nwith Trap Data" -> [w4515 _ w4549 w4588]
              tunnel: [w4515 w4530 w4549 w4588] -> w4419
              tunnel: w4418 -> [w4511 w4531 w4547 w4586]
              tunnel: w4417 -> [w4510 _ _ _]
              tunnel: [w4501 w4530 w4546 w4576] -> w4406
              tunnel: "Save Trap Pos. Data" -> [w4501 _ w4546 w4576]
              tunnel: w4409 -> [w4500 _ w4545 w4575]
              frame 1, Default {
                # "timeseries"
                n2788 = case shown="True" "Profile" {
                  tunnel: [w4524 w4528] -> w4505
                  tunnel: [w4524 w4527] -> w4504
                  tunnel: [w4524 w4526] -> w4503
                  tunnel: [w4524 w4525] -> w4502
                  frame False {
                    w4524 = 0.0 ("f")
                  }
                  frame True {
                    n2789 = local read "Current Position"() -> (w4529:cluster{dbl, dbl, dbl})
                    n2790 = local read "Y change (mm)"() -> (w4525:dbl)
                    n2791 = Unbundle(w4529) -> (w4528:dbl, w4527:dbl, w4526:dbl)
                  }
                }
                n2792 = local read "Save ave N"() -> (w4523:dbl)
                n2793 = Multiply(x=w4523, y=w4516) -> (x*y=w4522:dbl)
                n2794 = To Double Precision Float(number=w4500) -> (double precision float=w4514:dbl)
                n2795 = Build Array(w4511, w4516, w4522, w4521, w4520, 0.0 ("f")) -> (w4519:dbl[])
                n2796 = Build Array(w4514, w4505, w4504, w4503, w4502) -> (w4512:dbl[])
                n2797 = Select(t=u32 4000000000, s=w4510, f="N sets to save") -> (s? t:f=w4508:u32)
                n2798 = Build Array (concatenate)(w4519, w4518, w4512) -> (w4517:dbl[])
              }
              frame 2 {
                w4533 = 0.0 ("f")
                w4530 = FALSE ("Save APD Data\nwith Trap Data")
                # "calibration"
                n2799 = Boolean To (0,1)(Boolean=w4530) -> (0, 1=w4535:i16)
                n2800 = To Double Precision Float(number=w4535) -> (double precision float=w4534:dbl)
                n2801 = Build Array(w4534, w4533, w4533, w4533, w4533) -> (w4532:dbl[])
                n2802 = Build Array(w4531, w4536, w4536, w4543, w4542, 1.0 ("t")) -> (w4540:dbl[])
                n2803 = Build Array (concatenate)(w4540, w4539, w4532) -> (w4538:dbl[])
                "Calibrating Trap..." <- TRUE ("Calibrating...")
              }
              frame 4 {
                w4550 = 0.0 ("f")
                # "scan dir (x/y = 0/1)"
                # "cycles/step"
                # "n scans (f/b)"
                # "steps"
                # "freq. range"
                # "AOD raster scan"
                n2804 = local read "Number of F/B Scans (AOD)"() -> (w4557:u16)
                n2805 = local read "Cycles/step (AOD)"() -> (w4559:u64)
                n2806 = local read "Scan Range (MHz)"() -> (w4562:dbl)
                n2807 = local read "Scan steps (AOD)"() -> (w4561:u64)
                n2808 = local read "Scan BD"() -> (w4569:bool)
                n2809 = local read "Save ave N"() -> (w4574:dbl)
                n2810 = Boolean To (0,1)(Boolean=w4569) -> (0, 1=w4568:i16)
                n2811 = To Double Precision Float(number=w4557) -> (double precision float=w4556:dbl)
                n2812 = To Double Precision Float(number=w4561) -> (double precision float=w4560:dbl)
                n2813 = To Double Precision Float(number=w4559) -> (double precision float=w4558:dbl)
                n2814 = To Double Precision Float(number=w4568) -> (double precision float=w4567:dbl)
                n2815 = Multiply(x=w4574, y=w4552) -> (x*y=w4573:dbl)
                n2816 = To Double Precision Float(number=w4545) -> (double precision float=w4551:dbl)
                n2817 = Build Array(w4551, w4550, w4550, w4550, w4550) -> (w4548:dbl[])
                n2818 = local read "N sets should be saved"() -> (w4554:dbl)
                n2819 = Build Array(w4567, w4562, w4560, w4558, w4556) -> (w4564:dbl[])
                n2820 = Build Array(w4547, w4552, w4573, w4572, w4571, 2.0 ("t")) -> (w4566:dbl[])
                n2821 = Round Toward +Infinity(x=w4554) -> (ceil(x): smallest int >= x=w4555:dbl)
                n2822 = Build Array (concatenate)(w4566, w4565, w4548, w4564) -> (w4563:dbl[])
                n2823 = To Unsigned Long Integer(number=w4555) -> (unsigned 32bit integer=w4553:u32)
              }
              frame 8 {
                w4583 = 0.0 ("f")
                # "MCL raster scan"
                n2824 = local read "Number of scans (MCL)"() -> (w4578:u64)
                n2825 = local read "Scan lines (y)"() -> (w4577:u64)
                n2826 = local read "2D or 1D Scan"() -> (w4580:bool)
                n2827 = local read "Scan Range (V)\n(of steps)"() -> (w4599:dbl)
                n2828 = local read "Fast Scan Dir"() -> (w4606:bool)
                n2829 = local read "Cycles/step (MCL)"() -> (w4596:u64)
                n2830 = local read "Scan steps (MCL)"() -> (w4598:u64)
                n2831 = Select(t=w4577, s=w4580, f=w4578) -> (s? t:f=w4579:u64)
                n2832 = Boolean To (0,1)(Boolean=w4580) -> (0, 1=w4582:i16)
                n2833 = local read "Save ave N"() -> (w4611:dbl)
                n2834 = local read "Initial X"() -> (w4585:dbl)
                n2835 = local read "Initial Y"() -> (w4584:dbl)
                n2836 = To Double Precision Float(number=w4582) -> (double precision float=w4581:dbl)
                n2837 = Boolean To (0,1)(Boolean=w4606) -> (0, 1=w4605:i16)
                n2838 = To Double Precision Float(number=w4579) -> (double precision float=w4594:dbl)
                n2839 = To Double Precision Float(number=w4598) -> (double precision float=w4597:dbl)
                n2840 = To Double Precision Float(number=w4596) -> (double precision float=w4595:dbl)
                n2841 = To Double Precision Float(number=w4605) -> (double precision float=w4604:dbl)
                n2842 = Multiply(x=w4611, y=w4590) -> (x*y=w4610:dbl)
                n2843 = To Double Precision Float(number=w4575) -> (double precision float=w4589:dbl)
                n2844 = local read "N sets should be saved (MCL)"() -> (w4592:dbl)
                n2845 = Build Array(w4589, w4581, w4583, w4583, w4583) -> (w4587:dbl[])
                n2846 = Build Array(w4604, w4599, w4597, w4595, w4594, w4585, w4584) -> (w4601:dbl[])
                n2847 = Build Array(w4586, w4590, w4610, w4609, w4608, 3.0 ("t")) -> (w4603:dbl[])
                n2848 = Round Toward +Infinity(x=w4592) -> (ceil(x): smallest int >= x=w4593:dbl)
                n2849 = Build Array (concatenate)(w4603, w4602, w4587, w4601) -> (w4600:dbl[])
                n2850 = To Unsigned Long Integer(number=w4593) -> (unsigned 32bit integer=w4591:u32)
              }
            }
            n2851 = local read "Index"() -> (w4449:dbl)
            n2852 = call "Create new save file.vi"("Insert"="", "Ext"=".dat", "Index In"=w4449) -> ("Path Out"=w4408:path, "Index Out"=w4421:dbl)
            n2853 = local write "Save file name"(w4408) -> ()
            n2854 = local write "Index"(w4421) -> ()
            n2855 = local write "Save index"(w4421) -> ()
            n2856 = Array Size(array=w4432) -> (size(s)=w4433:i32)
            n2857 = Open/Create/Replace File(file path (use dialog)=w4408, operation (0:open)=T26."create", access (0:read/write)=enum16{"read/write", "read-only", "write-only"}."write-only") -> (refnum out=w4446:refnum<file>)  [unwired: 1 in, 4 out]
            n2858 = local write "Saving..."(TRUE ("Saving...")) -> ()
            n2859 = To Double Precision Float(number=w4433) -> (double precision float=w4431:dbl)
            n2860 = String Length(string="Comment (data description)") -> (length=w4429:i32)
            n2861 = To Double Precision Float(number=w4429) -> (double precision float=w4428:dbl)
            n2862 = Deny Access(7:w4446) -> (3:w4445:refnum<file>)  [unwired: 1 in, 2 out]
            n2863 = Build Array (concatenate)(w4431, w4432, w4428) -> (w4430:dbl[])
            n2864 = case "If fluorescence data to be saved" shown="True" w4419 {
              tunnel: w4408 -> [_ w4499]
              tunnel: [refnum<k0> refnum w4479] -> w4420
              frame False {
              }
              frame True {
                w4478 = 0.0
                n2865 = local read "APD Integration Time (s)"() -> (w4484:dbl)
                n2866 = local read "N APD Samp/step"() -> (w4477:dbl)
                n2867 = local read "Number of APDs"() -> (w4476:u8)
                n2868 = Path To String(path=w4499) -> (string=w4498:string)
                n2869 = String Length(string=w4498) -> (length=w4497:i32)
                n2870 = Subtract(x=w4497, y=4) -> (x-y=w4495:i32)
                n2871 = String Subset(string=w4498, length (rest)=w4495) -> (substring=w4494:string)  [unwired: 1 out]
                n2872 = Build Array(w4484, w4477, w4476, w4478, w4478, w4478, w4478, w4478) -> (w4481:dbl[])
                n2873 = Concatenate Strings(w4494, "_fl.dat" ("string")) -> (w4492:string)
                n2874 = Array Size(array=w4481) -> (size(s)=w4483:i32)
                n2875 = String To Path(string=w4492) -> (path=w4488:path)
                n2876 = Open/Create/Replace File(file path (use dialog)=w4488, operation (0:open)=T26."create", access (0:read/write)=enum16{"read/write", "read-only", "write-only"}."write-only") -> (refnum out=w4489:refnum<file>)  [unwired: 1 in, 4 out]
                n2877 = Deny Access(7:w4489) -> (3:w4485:refnum<file>)  [unwired: 1 in, 2 out]
                n2878 = To Double Precision Float(number=w4483) -> (double precision float=w4482:dbl)
                n2879 = Build Array (concatenate)(w4482, w4481) -> (w4480:dbl[])
                n2880 = Write to Binary File(file (use dialog)=w4485, data=w4480, 5:FALSE ("prepend array or string size? (T)"), 9:T25."big-endian, network order" ("byte order (0:big-endian, network order)")) -> (refnum out=w4479:refnum<file>)  [unwired: 1 in, 3 out]
              }
            }
            n2881 = case shown="True" w4406 {
              tunnel: w4408 -> [_ w4460]
              tunnel: [refnum<k0> refnum w4459] -> w4407
              frame False {
              }
              frame True {
                w4455 = 0.0 ("element")
                n2882 = Path To String(path=w4460) -> (string=w4474:string)
                n2883 = Build Array(w4455, w4455, w4455, w4455, w4455, w4455, w4455, w4455) -> (w4456:dbl[])
                n2884 = String Length(string=w4474) -> (length=w4473:i32)
                n2885 = Subtract(x=w4473, y=4) -> (x-y=w4471:i32)
                n2886 = Array Size(array=w4456) -> (size(s)=w4458:i32)
                n2887 = String Subset(string=w4474, length (rest)=w4471) -> (substring=w4470:string)  [unwired: 1 out]
                n2888 = To Double Precision Float(number=w4458) -> (double precision float=w4457:dbl)
                n2889 = Concatenate Strings(w4470, "_pos.dat" ("string")) -> (w4468:string)
                n2890 = Build Array (concatenate)(w4457, w4456) -> (w4454:dbl[])
                n2891 = String To Path(string=w4468) -> (path=w4464:path)
                n2892 = Open/Create/Replace File(file path (use dialog)=w4464, operation (0:open)=T26."create", access (0:read/write)=enum16{"read/write", "read-only", "write-only"}."write-only") -> (refnum out=w4465:refnum<file>)  [unwired: 1 in, 4 out]
                n2893 = Deny Access(7:w4465) -> (3:w4461:refnum<file>)  [unwired: 1 in, 2 out]
                n2894 = Write to Binary File(file (use dialog)=w4461, data=w4454, 5:FALSE ("prepend array or string size? (T)"), 9:T25."big-endian, network order" ("byte order (0:big-endian, network order)")) -> (refnum out=w4459:refnum<file>)  [unwired: 1 in, 3 out]
              }
            }
            n2895 = Write to Binary File(file (use dialog)=w4445, data=w4430, 5:w4426, 9:w4424) -> (refnum out=w4427:refnum<file>)  [unwired: 1 in, 3 out]
            n2896 = Write to Binary File(file (use dialog)=w4427, data="Comment (data description)", 5:w4426, 9:w4424) -> (refnum out=w4423:refnum<file>)  [unwired: 1 in, 3 out]
          }
        }
        n2897 = feedback-in #27(w4366) -> ()
        n2898 = feedback-in #28(w4393) -> ()
        n2899 = feedback-in #29(w4365) -> ()
        n2900 = feedback-in #30(w4376) -> ()
        n2901 = feedback-in #31(w4379) -> ()
        n2902 = feedback-in #32(w4392) -> ()
        n2903 = feedback-in #33(w4382) -> ()
      }
      frame #1 {
        n2904 = local read "Saving..."() -> (w4625:bool)
        n2905 = case shown="True" w4625 {
          tunnel: w4629 -> [_ w4640]
          tunnel: w4628 -> [_ w4654]
          tunnel: w4627 -> [_ w4650]
          tunnel: w4626 -> [_ w4649]
          tunnel: w4624 -> [_ w4648]
          tunnel: w4623 -> [_ w4643]
          tunnel: w4622 -> [_ w4642]
          tunnel: w4621 -> [_ w4641]
          tunnel: w4620 -> [_ w4639]
          tunnel: w4619 -> [_ w4637]
          tunnel: w4618 -> [_ w4636]
          tunnel: w4617 -> [_ w4635]
          tunnel: w4616 -> [_ w4634]
          tunnel: w4615 -> [_ w4633]
          tunnel: w4614 -> [_ w4632]
          tunnel: w4613 -> [_ w4631]
          tunnel: w4612 -> [_ w4630]
          frame False {
          }
          frame True {
            n2906 = Multiply(x=w4640, y=w4639) -> (x*y=→"Time (s)":dbl)
            n2907 = Less Or Equal?(x=w4640, y=w4648) -> (x <= y?=w4652:bool)
            n2908 = Or(x="Stop Saving", y="Abort save 2") -> (x .or. y?=w4644:bool)
            n2909 = Not(x=w4644) -> (.not. x?=w4653:bool)
            n2910 = And(x=w4652, y=w4653) -> (x .and. y?=w4651:bool)
            n2911 = case shown="True" w4651 {
              tunnel: w4654 -> [w4661 w4752]
              tunnel: [0.0 w4755] -> w4647
              tunnel: w4640 -> [_ w4753]
              tunnel: w4648 -> [_ w4754]
              tunnel: w4650 -> [_ w4749]
              tunnel: w4649 -> [_ _]
              tunnel: w4643 -> [w4659 w4742]
              tunnel: w4642 -> [w4658 w4743]
              tunnel: w4641 -> [_ w4741]
              tunnel: w4637 -> [_ w4740]
              tunnel: w4636 -> [_ w4664]
              tunnel: w4635 -> [_ w4733]
              tunnel: w4634 -> [_ w4680]
              tunnel: w4633 -> [w4655 w4697]
              tunnel: w4632 -> [w4656 w4696]
              tunnel: w4631 -> [_ w4693]
              tunnel: w4630 -> [_ w4691]
              frame False {
                w4657 = FALSE
                n2912 = Close File(refnum=w4661) -> ()  [unwired: 1 in, 2 out]
                n2913 = case shown="True" w4658 {
                  tunnel: w4659 -> [_ w4663]
                  frame False {
                  }
                  frame True {
                    n2914 = Close File(refnum=w4663) -> ()  [unwired: 1 in, 2 out]
                  }
                }
                n2915 = case shown="True" w4655 {
                  tunnel: w4656 -> [_ w4662]
                  frame False {
                  }
                  frame True {
                    n2916 = Close File(refnum=w4662) -> ()  [unwired: 1 in, 2 out]
                  }
                }
                n2917 = local write "Raster Scanning..."(w4657) -> ()
                n2918 = local write "Calibrating Trap..."(w4657) -> ()
                n2919 = call <vilib>:"Beep.vi"() -> ()  [unwired: 3 in, 9 out]
                n2920 = local write "Stop Saving"(w4657) -> ()
                "Saving..." <- w4657
              }
              frame True {
                n2921 = local read "Calibrating Trap..."() -> (w4744:bool)
                n2922 = case "Write fl. data" shown="True" w4743 {
                  tunnel: w4742 -> [_ w4778]
                  tunnel: w4741 -> [_ w4777]
                  frame False {
                  }
                  frame True {
                    n2923 = Write to Binary File(file (use dialog)=w4778, data=w4777, 5:FALSE ("prepend array or string size? (T)"), 9:T25."big-endian, network order" ("byte order (0:big-endian, network order)")) -> ()  [unwired: 1 in, 4 out]